vi "ADIS16448 IMU Example.vi"() -> ()   [LabVIEW 2018]
doc: "SimpleGyro Example\n\nThis example shows how to use a SimpleGyro sensor connected to the SPI port on the RoboRIO.\n\nThis example expects a USB cable connected from your development PC to the Type B USB Jack (next to the power input) on the roboRIO."
uses:
  <vilib>/Rock Robotics/WPI/ThirdParty/Sensors/ADIS16448 IMU/ADIS16448_IMU.lvlib
panel:
  in  "Calibrate On Open?":bool=TRUE
  out "IMU Angle Delta":cluster{"X":dbl, "Y":dbl, "Z":dbl} {"X" scale=-180.0..180.0; "Y" scale=-180.0..180.0; "Z" scale=-180.0..180.0}
  out "IMU AHRS":cluster{"Pitch":dbl, "Roll":dbl, "Yaw":dbl} {"Roll" scale=-180.0..180.0; "Pitch" scale=-90.0..90.0}
  out "IMU Data Out":T1 {"X Accel (g)" format="%#_3g"; "Y Accel (g)" format="%#_3g"; "Z Accel (g)" format="%#_3g"}
  in  "AHRS Algorithm":enum16{"Complementary", "Madgwick"}(ring)
  in  "AHRS Yaw Axis":enum16{"X", "Y", "Z"}(ring)=enum."Z"
  out "Sensor Ready?":bool
  out "IMU AHRS":cluster{"Pitch":dbl, "Roll":dbl, "Yaw":dbl}
  out "IMU Angle Delta":cluster{"X":dbl, "Y":dbl, "Z":dbl}
  in  "Reset Deltas?":bool
  out "Device Found?":bool
  in  "stop":bool
  # "FRC Analog Devices ADIS16448 IMU Example"
  # "Raw IMU Output Data"
  # "FRC ADI MXP Placement"
  # "Minimum LabVIEW version required: FRC 2019.0.0"
  # "Juan Chong -  Analog Devices Inc. - juan.chong@analog.com"
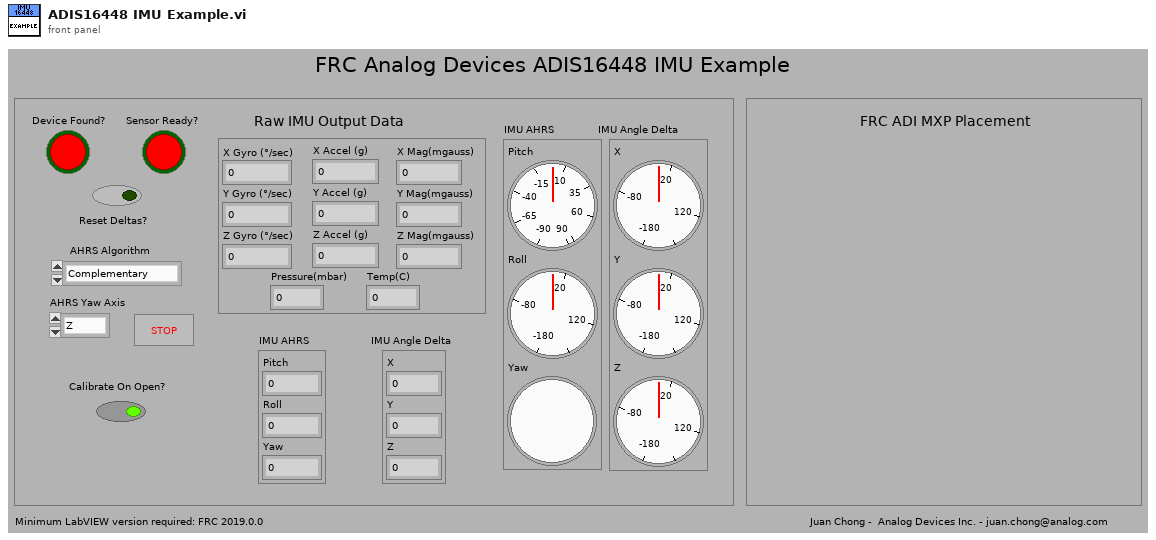
[diagram p1: front panel]
types:
  T1 = cluster{"X Gyro (°/sec)":dbl, "Y Gyro (°/sec)":dbl, "Z Gyro (°/sec)":dbl, "X Accel (g)":dbl, "Y Accel (g)":dbl, "Z Accel (g)":dbl, "X Mag(mgauss)":dbl, "Y Mag(mgauss)":dbl, "Z Mag(mgauss)":dbl, "Pressure(mbar)":dbl, "Temp(C)":dbl}
  T2 = typedef "ADIS16448_IMU.lvlib/ADI_IMU_ADIS16448_IMUDevRef.ctl" = cluster{"DevStatus":errorcluster, "Handle":i32, "SPI Bus":T3, "Device Found":bool, "Device Ready":bool, "Yaw Axis":enum16{"X", "Y", "Z"}, "AHRS Algorithm":enum16{"Complementary", "Madgwick"}, "Serial":u16, "Lot ID 2":u16, "Lot ID 1":u16, "Bytes Per Sample":u16, "Calibrate On Open?":bool}
  T3 = typedef "spi_bus.ctl" = enum16{"SPI On-Board, CS0", "SPI On-Board, CS1", "SPI On-Board, CS2", "SPI On-Board, CS3", "SPI MXP", "Invalid"}
  T4 = cluster{"X Angle":dbl, "Y Angle":dbl, "Z Angle":dbl}
  T5 = cluster{"X Gyro":dbl, "Y Gyro":dbl, "Z Gyro":dbl, "X Accel":dbl, "Y Accel":dbl, "Z Accel":dbl, "X Mag":dbl, "Y Mag":dbl, "Z Mag":dbl, "Pressure":dbl, "Temp":dbl}
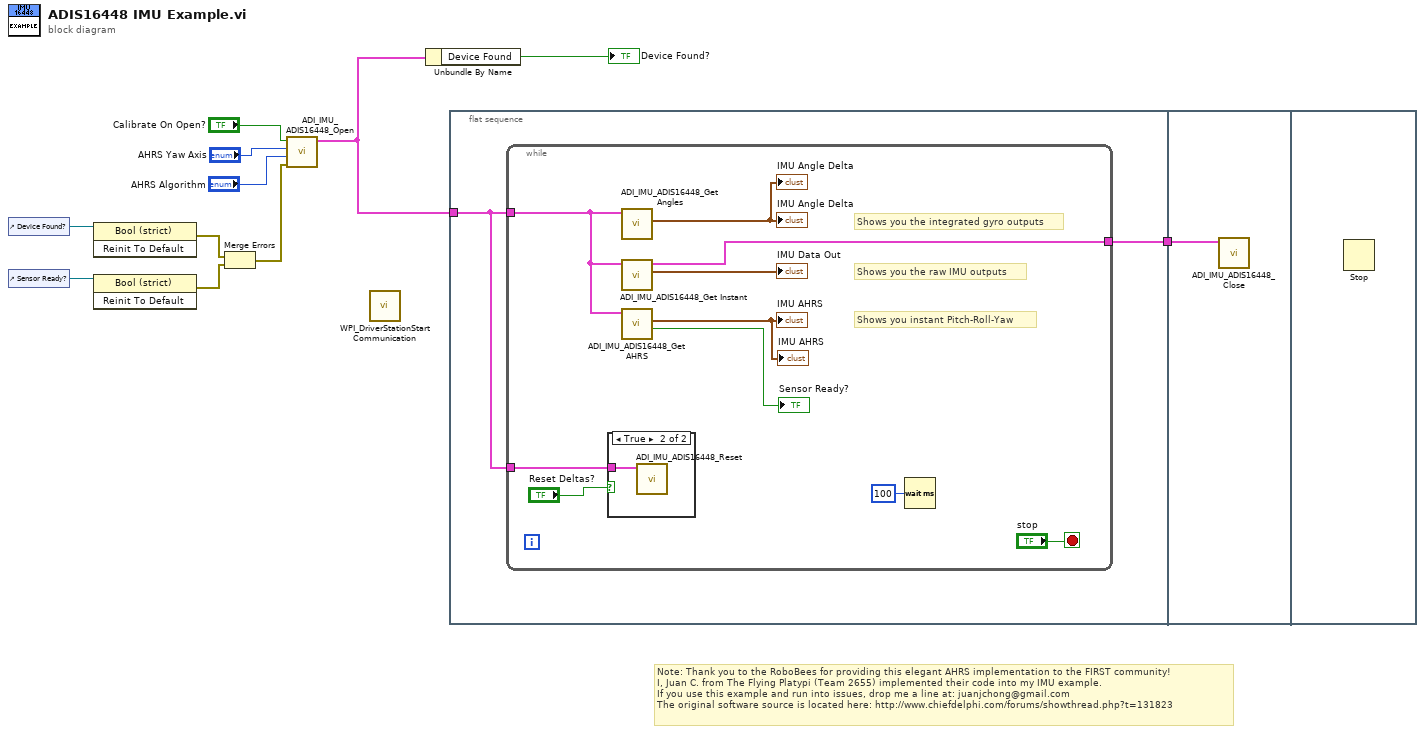
[diagram p0: block diagram]
diagram:
  # "Note: Thank you to the RoboBees for providing this elegant AHRS implementation to the FIRST community!\nI, Juan C. from The Flying Platypi (Team 2655) implemented their code into my IMU example.\nIf you use this example and run into issues, drop me a line at: juanjchong@gmail.com\nThe original software source is located here: http://www.chiefdelphi.com/forums/showthread.php?t=131823"
  n1 = control-ref of="Device Found?"() -> (w6:refnum<vi>)
  n2 = control-ref of="Sensor Ready?"() -> (w5:refnum<vi>)
  n3 = invoke class="Bool (strict)" method="Reinit To Default"(reference=w6) -> (error out=w4:errorcluster)  [unwired: 2 in, 2 out]
  n4 = invoke class="Bool (strict)" method="Reinit To Default"(reference=w5) -> (error out=w3:errorcluster)  [unwired: 2 in, 2 out]
  n5 = Merge Errors(w4, w3) -> (w2:errorcluster)
  n6 = call <vilib>:"ADI_IMU_ADIS16448_Open.vi"("error in"=w2, "AHRS Algorithm"="AHRS Algorithm", "Yaw Axis"="AHRS Yaw Axis", "Calibrate On Open"="Calibrate On Open?") -> ("ADI IMU DevRef Out"=w9:T2)  [unwired: 6 in, 1 out]
  n7 = call <vilib>:"WPI_DriverStationStart Communication.vi"() -> ()  [unwired: 12 in]
  n8 = Unbundle By Name(w9) -> ("Device Found"=→"Device Found?":bool)
  n9 = flat-sequence {
    tunnel: w9 -> [w13]
    tunnel: [w12] -> w8
    tunnel: w8 -> [w25]
    frame #0 {
      n10 = while {
        tunnel: w13 -> [w15]
        tunnel: w13 -> [w22]
        tunnel: [w16] -> w12
        stop <- "stop" stop-if-true
        # "Shows you the integrated gyro outputs"
        # "Shows you the raw IMU outputs"
        # "Shows you instant Pitch-Roll-Yaw"
        n11 = case shown="True" "Reset Deltas?" {
          tunnel: w22 -> [_ w24]
          frame False {
          }
          frame True {
            n12 = call <vilib>:"ADI_IMU_ADIS16448_Reset.vi"("ADI IMU DevRef"=w24) -> ()  [unwired: 9 in, 2 out]
          }
        }
        n13 = call <vilib>:"ADI_IMU_ADIS16448_Get Angles.vi"("ADI IMU DevRef"=w15) -> ("IMU Angles Out"=→"IMU Angle Delta" →"IMU Angle Delta":T4)  [unwired: 7 in, 3 out]
        n14 = call <vilib>:"ADI_IMU_ADIS16448_Get Instant.vi"("ADI IMU DevRef"=w15) -> ("IMU Data Out"=→"IMU Data Out":T5, "ADI IMU DevRef Out"=w16:T2)  [unwired: 7 in, 2 out]
        n15 = call <vilib>:"ADI_IMU_ADIS16448_Get AHRS.vi"("ADI IMU DevRef"=w15) -> ("Sensor Ready Out"=→"Sensor Ready?":bool, "IMU AHRS Out"=→"IMU AHRS" →"IMU AHRS":cluster{"Pitch":dbl, "Roll":dbl, "Yaw":dbl})  [unwired: 7 in, 2 out]
        n16 = Wait (ms)(milliseconds to wait=u32 100) -> ()  [unwired: 1 out]
      }
    }
    frame #1 {
      n17 = call <vilib>:"ADI_IMU_ADIS16448_Close.vi"("ADI IMU DevRef"=w25) -> ()  [unwired: 10 in, 1 out]
    }
    frame #2 {
      n18 = Stop() -> ()  [unwired: 1 in]
    }
  }
